vi "UHR-Fleezers Control (host) - 10.2.vi"() -> ()   [LabVIEW 2009] (continued)
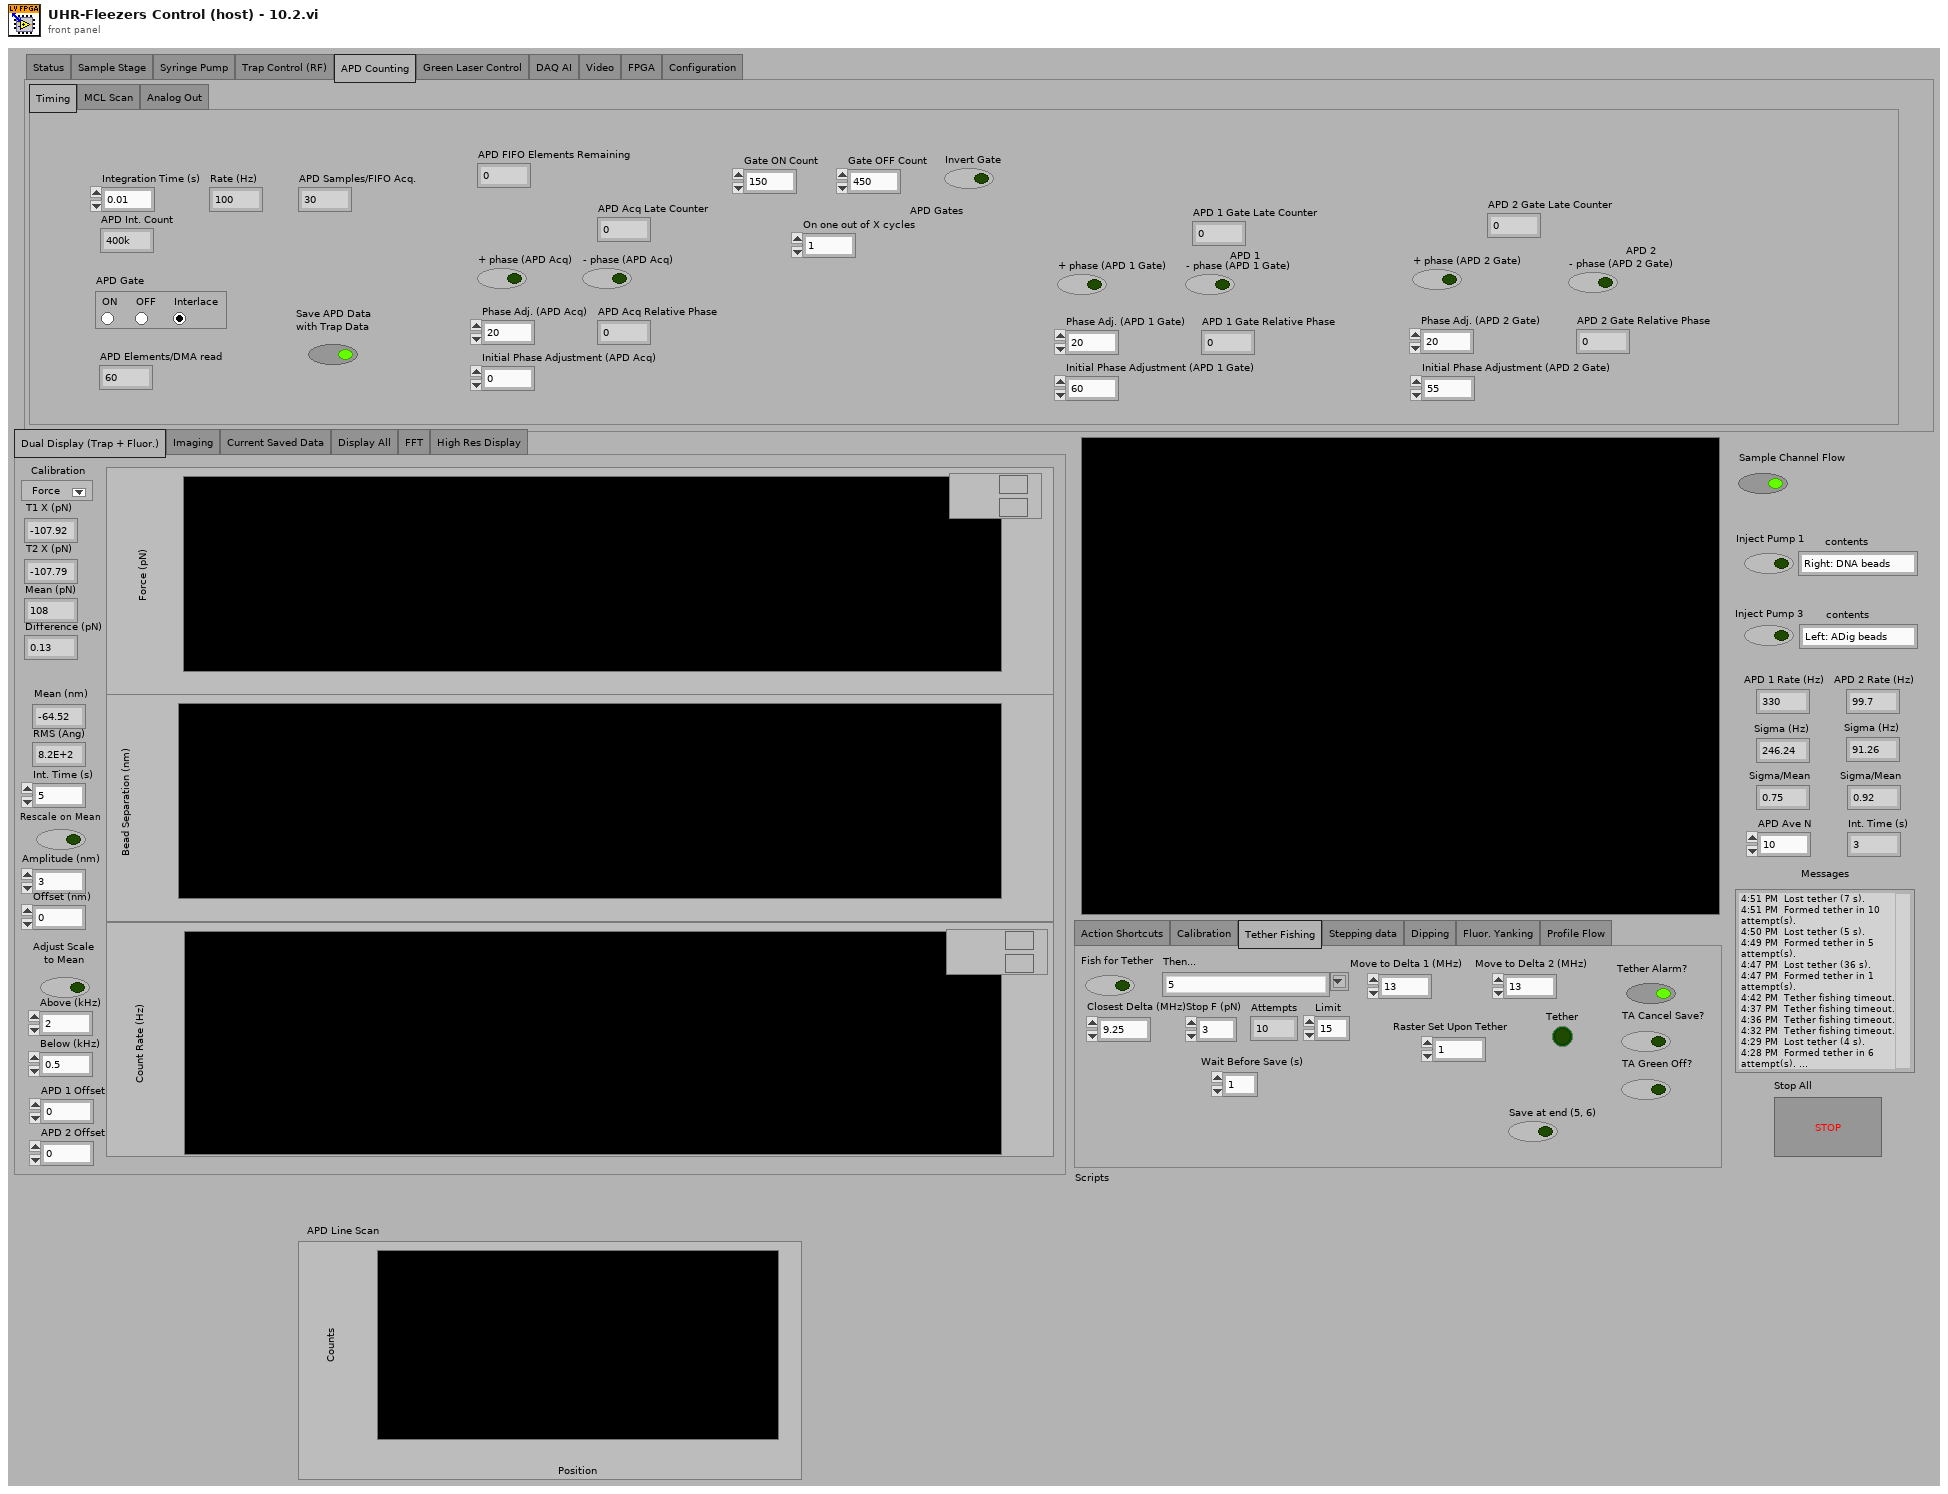
[diagram p1: front panel]
types:
  T1 = enum32{"Action Shortcuts", "Calibration", "Tether Fishing", "Stepping data", "Dipping", "Fluor. Yanking", "Profile Flow"}
  T2 = typedef "IMAQ Image.ctl" = refnum<image>
  T3 = enum32{"Dual Display (Trap + Fluor.)", "Imaging", "Current Saved Data", "Display All", "FFT", "High Res Display"}
  T4 = enum32{"Status", "Sample Stage", "Syringe Pump", "Trap Control (RF)", "APD Counting", "Green Laser Control", "DAQ AI", "Video", "FPGA", "Configuration"}
  T5 = cluster{"Pump 1":cluster{"Diameter (mm)":dbl, "Units":dbl, "Volume":dbl, "Rate":dbl}, "Pump 2":cluster{"Diameter (mm)":dbl, "Units":dbl, "Volume":dbl, "Rate":dbl}, "Pump 3":cluster{"Diameter (mm)":dbl, "Units":dbl, "Volume":dbl, "Rate":dbl}}
  T6 = enum32{"IR Laser Interlacing (Direct RF Board Control Method)", "AOD Raster Scan", "Feedback on Trap Intensity", "Feedback on Trap Position"}
  T7 = typedef "LVPoint32TypeDef.ctl" = cluster{"Horizontal":i32, "Vertical":i32}
  T8 = cluster{"Scan Range AOD (nm) 2":dbl, "Step Size AOD (nm) 2":dbl, "Scan Speed AOD (nm/s) 2":dbl, "Number of scans (AOD) 2":u16, "Label":string}[]
  T9 = cluster{"Set 1":cluster{"proportional gain (Kc)":i16, "integral gain (Kc*Ts/Ti)":i16, "derivative gain (Kc*Td/Ts)":i16}, "Set 2":cluster{"proportional gain (Kc)":i16, "integral gain (Kc*Ts/Ti)":i16, "derivative gain (Kc*Td/Ts)":i16}}
  T10 = cluster{"Trap 1":fxp<+/-,16,1>, "Trap 2":fxp<+/-,16,1>}
  T11 = cluster{"proportional gain (Kc)":fxp<+/-,16,8>, "integral gain (Kc*Ts/Ti)":fxp<+/-,16,8>, "derivative gain (Kc*Td/Ts)":fxp<+/-,16,8>}
  T12 = cluster{"output high":fxp<+/-,16,1>, "output low":fxp<+/-,16,1>}
  T13 = cluster{"Set 1":fxp<+/-,16,1>, "Set 2":fxp<+/-,16,1>}
  T14 = cluster{"proportional gain (Kc)":i16, "integral gain (Kc*Ts/Ti)":i16, "derivative gain (Kc*Td/Ts)":i16}
  T15 = cluster{"Set 1":bool, "Set 2":bool, "Set 3":bool}
  T16 = typedef "LVMinMaxIncTypeDef.ctl" = cluster{"Minimum":dbl, "Maximum":dbl, "Increment":dbl}
  T17 = typedef "Image Type" = u32
  T18 = typedef "nirio_resource_hc.ctl" = tag
  T19 = typedef "niFpgaNodeNameForErrorReporting.ctl" = enum16{"Open FPGA VI Reference", "Read/Write Control", "Invoke Method: Abort", "Invoke Method: Acknowledge IRQ", "Invoke Method: Download", "Invoke Method: FIFO.Configure", "Invoke Method: FIFO.Read", "Invoke Method: FIFO.Start", "Invoke Method: FIFO.Stop", "Invoke Method: FIFO.Write", "Invoke Method: Reset", "Invoke Method: Run", "Invoke Method: Wait on IRQ", "Close FPGA VI Reference"}
  T20 = typedef "niLvFpgaWhatHappensToTopLevelVI.ctl" = enum16{"top level VI scripted behind XNode", "top level VI inlined behind XNode"}
  T21 = typedef "openfpgaref.8.6.ctl" = refnum<k20>
  T22 = cluster{"New Image":T2, "New Image":T2, "New Image":T2, "New Image":T2}
  T23 = typedef "XDNodeRunTimeDep.lvlib/timing_clust.ctl" = cluster{"Expected End [f-1]":u64, "Actual End [f-1]":u64, "Finished Late? [f-1]":bool, "Expected End [i-1]":u64, "Actual End [i-1]":u64, "Finished Late? [i-1]":bool, "Expected Start [i]":u64, "Actual Start [i]":u64, "Expected Start [f]":u64, "Actual Start [f]":u64, "Source Name":string, "Structure Name":string, "Period":i64, "Deadline":i64, "Offset":i64, "Start":i64, "Priority":i32, "Timeout":i32, "Mode":T24, "Wakeup Reason":T25, "Error":errorcluster, "Source Type":string, "Secondary Source Type":string, "Global End Time":u64, "Global Start Time":u64, "Frame Duration":u64, "Iteration Duration":u64, "Assigned CPU":i32, "I/O Scan Engine Mode":u32}
  T24 = typedef "XDNodeRunTimeDep.lvlib/nitl_modes.ctl" = enum32{"No Change", "Process missed periods, maintain original phase", "Discard missed periods, maintain original phase", "Process missed periods, ignore original phase", "Discard missed periods, ignore original phase"}
  T25 = typedef "XDNodeRunTimeDep.lvlib/wakeup.ctl" = enum32{"Normal", "Aborted", "Asynchronous wakeup", "Timing source error", "Timed loop error", "Timeout"}
  T26 = enum32{"Normal Display", "Dual Display (APD)", "FFT", "High Res Display"}
  T27 = cluster{"Origin Pixel":cluster{"X":sgl, "Y":sgl}, "Angle Relative to Horizontal (deg)":sgl, "Axis Reference":u32}
  T28 = typedef "Simple Grid Descriptor" = cluster{"X Step":sgl, "Y Step":sgl, "Unit":T29}
  T29 = typedef "Image Unit" = enum32{"Undefined", "Angström", "Micrometer", "Millimeter", "Centimeter", "Meter", "Kilometer", "Microinch", "Inch", "Feet", "Nautical miles", "Standard miles", "Steps"}
  T30 = cluster{"averaging mode":u16, "weighting mode":u16, "number of averages":u32}
  T31 = cluster{"dB On (F)":bool, "unwrap phase (F)":bool, "convert to degree (F)":bool}
  T32 = cluster{"Green FB Ch 0":i16, "Green FB Ch 1":i16, "Green FB Ch 2":i16}
  T33 = enum16{"open", "replace", "create", "open or create", "replace or create", "replace or create with confirmation"}
  T34 = enum16{"big-endian, network order", "native, host order", "little-endian"}
  T35 = cluster{string, string, string, string, string, string, string, string}
  T36 = cluster{string, string, string, string, string, string, string, string, string, string, string, string}
  T37 = cluster{string, string, string, string, string, string, string, string, string, string, string, string, string}
  T38 = cluster{string, string, string, string, string, string, string, string, string, string, string, string, string, string}
  T39 = cluster{"BD 1 Frequency 1 (MHz)":dbl, "BD 1 Frequency 2 (MHz)":dbl}
  T40 = cluster{"f0":dbl, "df":dbl, "magnitude":dbl[]}[][]
  T41 = cluster{"Green FB Ch 0":dbl, "Green FB Ch 1":dbl, "Green FB Ch 2":dbl}
  T42 = cluster{"Scan Range AOD (nm) 2":dbl, "Step Size AOD (nm) 2":dbl, "Scan Speed AOD (nm/s) 2":dbl, "Number of scans (AOD) 2":u16, "Label":string}
  T43 = cluster{"[0]":dbl, "[1]":dbl, "[2]":dbl, "[3]":dbl, "[4]":dbl, "[5]":dbl}
  T44 = cluster{"Diameter (mm)":dbl, "Units":dbl, "Volume":dbl, "Rate":dbl}
  T45 = cluster{"Left":i32, "Top":i32, "Width":u32, "Height":u32}
  T46 = cluster{cluster{"Left":i32, "Top":i32, "Width":u32, "Height":u32}}[]
  T47 = enum32{"setting", "request", "request control", "info", "statistics", "system settings", "I/O sub system", "HRT control", "camera descriptions", "device specific data", "event sub system settings", "event sub system results", "image memory manager"}
  T48 = typedef "AviRefnum.ctl" = refnum<k1>
  T49 = typedef "imagedata.ctl" = cluster{"image type":i32, "image depth":i32, "image":u8[], "mask":u8[], "colors":u32[], "Rectangle":cluster{"left":i16, "top":i16, "right":i16, "bottom":i16}}
diagram:
  w25 = u16 20 items=["1.0"=10, "1.5"=15, "2.0"=20] ("stop bits (10: 1 bit)")
  w32 = T17 2 items=["Grayscale (U8)", "Grayscale (I16)", "Grayscale (SGL)", "Complex (CSG)", "RGB (U32)", "HSL (U32)", "RGB (U64)", "Grayscale (U16)"] ("Image Type")
  w100 = cluster{"output high":i16, "output low":i16} {"output high"=3000, "output low"=0} ("FB output range 1")
  w182 = 10.0 ("y")
  w181 = 32767.0 ("y")
  w197 = 6.0  # clock mult.
  w198 = 49152000.0  # TCXO frequ.
  n1 = Build Array("DIO count 1 (ticks)", "DIO count 2 (ticks)", "DIO count 3 (ticks)") -> (w87:u32[])
  n2 = Multiply(x="APD Integration Time (s)", y=40000000.0) -> (x*y=w107:dbl)
  n3 = Reciprocal(x="APD Integration Time (s)") -> (1/x=w104:dbl)
  n4 = local write "APD Acq Rate (Hz)"(w104) -> ()
  n5 = local read "AO1"() -> (w176:dbl)
  n6 = local read "AO2"() -> (w175:dbl)
  n7 = To Unsigned Long Integer(number=w107) -> (unsigned 32bit integer=w106:u32)
  "APD Int. Count" <- w106
  n8 = local read "Scan Increment (MHz)"() -> (w193:dbl)
  n9 = local read "Continuous MCL Scanning"() -> (w163:bool)
  n10 = local read "Fast Scan Dir"() -> (w162:bool)
  n11 = Multiply(x=w176, y=w181) -> (x*y=w178:dbl)
  n12 = local read "Number of scans (MCL)"() -> (w164:u64)
  n13 = Multiply(x=w175, y=w181) -> (x*y=w180:dbl)
  n14 = Divide(x=w178, y=w182) -> (x/y=w177:dbl)
  n15 = Divide(x=w180, y=w182) -> (x/y=w179:dbl)
  n16 = To Word Integer(number=w177) -> (16bit integer=w174:i16)
  n17 = To Word Integer(number=w179) -> (16bit integer=w173:i16)
  n18 = Not(x=w162) -> (.not. x?=w157:bool)
  n19 = local read "Cycles/step (MCL)"() -> (w165:u64)
  n20 = Multiply(x=w193, y=1000.0) -> (x*y=w200:dbl)
  n21 = local read "Scan steps (MCL)"() -> (w166:u64)
  n22 = local write "Trap Pos FIFO Timeout"(u16 0 ("Trap Pos FIFO Timeout")) -> ()
  n23 = local read "Desired Scan Incr (V)"() -> (w168:dbl)
  n24 = Scale By Power Of 2(n=48, x=w200) -> (x*2^n=w201:dbl)
  n25 = Multiply(x=w198, y=w197) -> (x*y=w196:dbl)
  n26 = Divide(x=w201, y=w196) -> (x/y=w195:dbl)
  n27 = local read "Setpoints (V)"() -> (w215:cluster{"Set 1":dbl, "Set 2":dbl})
  n28 = property on="AI Count (ticks)" class="DigNum (strict)"("Val(Sgnl)"="AI Count (ticks)") -> ()  [unwired: 2 in, 2 out]
  n29 = local read "Number Interlace Sets"() -> (w80:u8)
  n30 = Split 1D Array(array=w87, index=w80) -> (first subarray=w89:u32[])  [unwired: 1 out]
  n31 = Add Array Elements(numeric array=w89) -> (sum=w88:u32)
  n32 = local read "# Samples/channel"() -> (w185:u32)
  n33 = To Quad Integer(1:w195) -> (0:w192:i64)
  n34 = local read "Number of F/B Scans (AOD)"() -> (w186:u16)
  n35 = local read "Not-Interlacing Set"() -> (w79:enum32{"Set 1", "Set 2", "Set 3"})
  n36 = To Unsigned Byte Integer(number=w79) -> (unsigned 8bit integer=w85:u8)
  n37 = Index Array(array=w87, index=w85) -> (element=w86:u32)
  n38 = Divide(x=40000000.0, y="AI Count (ticks)") -> (x/y=w153:dbl)
  n39 = Multiply(x=w168, y=32767.0) -> (x*y=w170:dbl)
  n40 = local read "Feedback On/Off"() -> (w218:cluster{"Set 1":bool, "Set 2":bool})
  n41 = local read "PID Gains"() -> (w210:T9)
  n42 = local read "Scan steps (AOD)"() -> (w191:u64)
  n43 = local read "All FB On/Off"() -> (w219:bool)
  n44 = local read "Cycles/step (AOD)"() -> (w190:u64)
  n45 = local write "AI rate (Hz)"(w153) -> ()
  n46 = Divide(x=w170, y=10.0) -> (x/y=w169:dbl)
  n47 = Multiply(x=w191, y=w190) -> (x*y=w189:u64)
  n48 = Multiply(x=3276.7, y=w215) -> (x*y=w214:cluster{"Set 1":dbl, "Set 2":dbl})
  n49 = To Word Integer(number=w169) -> (16bit integer=w167:i16)
  n50 = Multiply(x=w189, y=u64 2) -> (x*y=w187:u64)
  n51 = Divide(x=w153, y="FPGA Ave.") -> (x/y=w154:dbl)
  n52 = To Word Integer(number=w214) -> (16bit integer=w213:cluster{"Set 1":i16, "Set 2":i16})
  n53 = xnode "Open FPGA VI Reference"("resource name"=T18 "750kHzDAQ") -> ("FPGA VI Reference Out"=w207:refnum<k20>, "error out"=w206:errorcluster)  [unwired: 1 in]
  n54 = local read "Sets to FIFO (Traps)"() -> (w222:T15)
  n55 = Unbundle By Name(w210) -> ("Set 1"=w209:T14, "Set 2"=w208:T14)
  n56 = Multiply(x=w187, y=w186) -> (x*y=w184:u64)
  n57 = Divide(x=w184, y=w185) -> (x/y=w183:dbl)
  n58 = local write "Ave. Rate (Hz)"(w154) -> ()
  n59 = Unbundle By Name(w213) -> ("Set 1"=w212:i16, "Set 2"=w211:i16)
  n60 = local read "2D or 1D Scan"() -> (w101:bool)
  n61 = local write "Data points/scans"(w184) -> ()
  n62 = And(x=w218, y=w219) -> (x .and. y?=w217:cluster{"Set 1":bool, "Set 2":bool})
  n63 = local read "Scan BD"() -> (w202:bool)
  n64 = Reciprocal(x=w154) -> (1/x=w155:dbl)
  n65 = local write "Data points/scan (f/b)"(w187) -> ()
  n66 = local read "N Acq Sets (Traps + Fl.)"() -> (w146:i16)
  n67 = local write "N sets should be saved"(w183) -> ()
  n68 = Unbundle By Name(w217) -> ("Set 1"=w221:bool, "Set 2"=w220:bool)
  n69 = xnode "Invoke Method"("FPGA VI Reference In"=w207, "error in"=w206) -> ("FPGA VI Reference Out"=w99:refnum<k20>, "error out"=w120:errorcluster)
  n70 = local read "Interlace"() -> (w81:bool)
  n71 = Select(t=w88, s=w81, f=w86) -> (s? t:f=w78:u32)
  n72 = local write "Update Count (MCL)"(w78) -> ()
  n73 = local write "Total Counts (ticks)"(w78) -> ()
  n74 = local write "Ave. Period (s)"(w155) -> ()
  n75 = property on="2D or 1D Scan" class="Bool (strict)"("Val(Sgnl)"=w101) -> ()  [unwired: 2 in, 2 out]
  n76 = xnode "Read/Write Control"("FPGA VI Reference In"=w98, "error in"=w120, "ai count"="AI Count (ticks)", "Interlace ON/OFF"=w81, "Number Interlace Cycles"=w80, "AI1 Sets to FIFO"=w222, "FB On/Off Set 1"=w221, "FB On/Off Set 2"=w220, "Interlace Off Parameters"=w79, "FB Setpoint Set 1"=w212, "FB Setpoint Set 2"=w211, "FB Gains Set 1"=w209, "FB Gains Set 2"=w208, "FB output range 1"=w100, "FB output range 2"=w100, "Cycles per step"=w190, "Scan BD"=w202, "Number of scans"=w186, "Scan steps"=w191, "Scan freq.  increment"=w192, "AO1"=w174, "AO2"=w173, "Scan freq.  increment (MCL)"=w167, "Scan steps (MCL)"=w166, "Cycles per step (MCL)"=w165, "Number of scans (MCL)"=w164, "MCL count"=w78, "Cont. Scan (MCL)"=w163, "MCL Scan Axis"=w157, "1D or 2D Scan?"=w101, "N of AI1 Int Acq Sets"=w146, "Freq or Amp switch first"="Freq or Amp switch first", "Freq switch delay"="Freq switch delay", "Amp switch delay"="Amp switch delay", "Swap F1 and F2"="Swap F1 and F2", "APD Acq Rate Count"=w106, "APD to FIFO"=FALSE, "APD Gate Operating Mode"="APD Gate", "APD Gate ON Count"="APD Gate ON Count", "APD Gate OFF Count"="APD Gate OFF Count", "Invert APD Gate"="Invert APD Gate", "DIO count 1 (ticks)"="DIO count 1 (ticks)", "DIO count 2 (ticks)"="DIO count 2 (ticks)", "DIO count 3 (ticks)"="DIO count 3 (ticks)", "APD 1 AO scale factor"="APD 1 AO Mult.", "APD 2 AO scale factor"="APD 2 AO Mult.") -> ("FPGA VI Reference Out"=w73:refnum<k20>, "error out"=w75:errorcluster)  [unwired: 1 in]
  n77 = local read "Green Laser ON/Interlacing"() -> (w76:bool)
  n78 = local read "Green laser mode"() -> (w77:enum32{"Laser ON", "Laser OFF", "Interlace"})
  n79 = local read "GI Frequency, OFF count"() -> (w69:u32)
  n80 = local read "GI Frequency, ON count"() -> (w68:u32)
  n81 = Multiply(x="Current When FB OFF (%)", y=655.35) -> (x*y=w59:dbl)
  n82 = local read "Green FB Count"() -> (w67:u32)
  n83 = Multiply(x="Green FB Setpoint (mV)", y=3.2767) -> (x*y=w56:dbl)
  n84 = To Unsigned Word Integer(number=w59) -> (unsigned 16bit integer=w57:u16)
  n85 = local read "Invert GI"() -> (w71:bool)
  n86 = To Word Integer(number=w56) -> (16bit integer=w54:i16)
  n87 = case shown="False" w76 {
    tunnel: w77 -> [_ w248]
    tunnel: [enum32{"Laser ON", "Laser OFF", "Interlace"}."Laser OFF" ("Green laser mode") w248] -> w70
    frame #0 {
    }
    frame #1 {
    }
  }
  n88 = local read "Trap Pos. AI1 X Pre-scale"() -> (w11:u16)
  n89 = local read "Trap Pos FB Monitor\nT1 or T2"() -> (w18:bool)
  n90 = local read "Trap Pos FB Int Count"() -> (w4:u16)
  n91 = local read "Trap Pos FB Negate Action"() -> (w17:bool)
  n92 = local read "Trap Pos. FB Offset Factor"() -> (w16:i64)
  n93 = local read "Trap Pos. FB Mult Factor"() -> (w15:i64)
  n94 = local read "Trap Pos. FB Gains"() -> (w13:T11)
  n95 = local read "Trap Pos. FB Range"() -> (w14:T12)
  n96 = xnode "Read/Write Control"("FPGA VI Reference In"=w73, "error in"=w75, "Green interlace ON count 2"=w68, "Green interlace OFF count 2"=w69, "Invert GI 2"=w71, "Operating Mode 2"=w70, "Green FB Gains"="Green FB Gains", "Green FB Setpoint"=w54, "Green FB On/Off"="Green FB On/Off", "Current Out"=w57, "Green int current ON count adj"="Green int current ON count adj", "Green FB Count"=w67, "Operating Mode"=w70, "Green interlace OFF count"=w69, "Green interlace ON count"=w68, "Invert GI"=w71, "Trap Pos FB Monitor T1 or T2"=w18, "Trap Pos FB Negate Action"=w17, "Trap Pos. FB Offset Factor"=w16, "Trap Pos. FB Mult Factor"=w15, "Trap Pos. FB Range"=w14, "Trap Pos. FB Gains"=w13, "Force feedback"=FALSE, "AI1 X Scale"=w11, "Trap Pos to FIFO"=TRUE, "Trap Pos FB Int Count"=w4) -> ("FPGA VI Reference Out"=w72:refnum<k20>, "error out"=w74:errorcluster)
  n97 = xnode "Invoke Method"("FPGA VI Reference In"=w72, "error in"=w74, "Depth"="Trap AI FIFO Depth") -> ("FPGA VI Reference Out"=w21:refnum<k20>, "error out"=w20:errorcluster)
  n98 = xnode "Invoke Method"("FPGA VI Reference In"=w21, "error in"=w20, "Depth"="Trap Position FIFO Depth") -> ("FPGA VI Reference Out"=w6:refnum<k20>, "error out"=w5:errorcluster)
  n99 = flat-sequence {
    tunnel: w99 -> [w253]
    tunnel: [w253] -> w98
    tunnel: [w252] -> w97
    tunnel: [w251] -> w96
    tunnel: [w249] -> w94
    tunnel: [w250] -> w95
    frame #0 {
      w250 = T16 {"Minimum"=0.0, "Maximum"=40.0, "Increment"=1.0} ("Min Max Inc")
      w249 = T16 {"Minimum"=0.0, "Maximum"=50.0, "Increment"=1.0} ("Data Entry Limits")
      w252 = T16 {"Minimum"=60.0, "Maximum"=90.0, "Increment"=1.0} ("Min Max Inc")
      w251 = T16 {"Minimum"=0.0, "Maximum"=50.0, "Increment"=1.0} ("Data Entry Limits")
      n100 = property on="BD 2 Frequency 1 (MHz)" class="DigNum (strict)"("Data Range"=w250) -> ()  [unwired: 2 in, 2 out]
      n101 = property on="BD 2 Frequency 3 (MHz)" class="DigNum (strict)"("Data Range"=w250) -> ()  [unwired: 2 in, 2 out]
      n102 = property on="BD 2 Frequency 2 (MHz)" class="DigNum (strict)"("Data Range"=w250) -> ()  [unwired: 2 in, 2 out]
      n103 = property on="BD 1 Frequency 1 (MHz)" class="DigNum (strict)"("Data Range"=w252) -> ()  [unwired: 2 in, 2 out]
      n104 = property on="BD 1 Frequency 2 (MHz)" class="DigNum (strict)"("Data Range"=w252) -> ()  [unwired: 2 in, 2 out]
      n105 = property on="BD 1 Frequency 3 (MHz)" class="DigNum (strict)"("Data Range"=w252) -> ()  [unwired: 2 in, 2 out]
      n106 = property on="BD 2 Amplitude 1 (%)" class="DigNum (strict)"("Data Range"=w249) -> ()  [unwired: 2 in, 2 out]
      n107 = property on="BD 2 Amplitude 2 (%)" class="DigNum (strict)"("Data Range"=w249) -> ()  [unwired: 2 in, 2 out]
      n108 = property on="BD 2 Amplitude 3 (%)" class="DigNum (strict)"("Data Range"=w249) -> ()  [unwired: 2 in, 2 out]
      n109 = property on="BD 1 Amplitude 3 (%)" class="DigNum (strict)"("Data Range"=w251) -> ()  [unwired: 2 in, 2 out]
      n110 = property on="BD 1 Amplitude 2 (%)" class="DigNum (strict)"("Data Range"=w251) -> ()  [unwired: 2 in, 2 out]
      n111 = property on="BD 1 Amplitude 1 (%)" class="DigNum (strict)"("Data Range"=w251) -> ()  [unwired: 2 in, 2 out]
      "X RF Frequency Limits (MHz)" <- w252
      "X RF Amplitude Limits (%)" <- w251
      "Y RF Amplitude Limits (%)" <- w249
      "Y RF Frequency Limits (MHz)" <- w250
    }
  }
  n112 = xnode "Invoke Method"("FPGA VI Reference In"=w6, "error in"=w5) -> ("FPGA VI Reference Out"=w119:refnum<k20>, "error out"=w118:errorcluster)  [unwired: 1 out]
  n113 = flat-sequence "Initial FPGA Loop Relative Phase Adjustment" {
    tunnel: "Initial Phase Adjustment (AI1)" -> [w264]
    tunnel: "Initial Phase Adjustment (GI)" -> [w263]
    tunnel: w119 -> [w262]
    tunnel: w118 -> [w261]
    tunnel: "Initial Phase Adj. (MCL)" -> [w260]
    tunnel: [w265] -> w128
    tunnel: [w259] -> w124
    tunnel: "Initial Phase Adjustment (APD Acq)" -> [w258]
    tunnel: "Initial Phase Adjustment (APD 1 Gate)" -> [w257]
    tunnel: "Initial Phase Adjustment (Green FB)" -> [w256]
    tunnel: "Initial Phase Adjustment (GI) 2" -> [w255]
    tunnel: "Initial Phase Adjustment (APD 2 Gate)" -> [w254]
    tunnel: w128 -> [w436]
    tunnel: [w437] -> w125
    tunnel: w124 -> [w437]
    tunnel: [w436] -> w123
    tunnel: w125 -> [w440]
    tunnel: w123 -> [w439]
    tunnel: [w442] -> w122
    tunnel: [w441] -> w121
    tunnel: [w621] -> w126
    tunnel: [w622] -> w127
    tunnel: w122 -> [w622]
    tunnel: w121 -> [w621]
    frame #0 {
      n114 = xnode "Read/Write Control"("FPGA VI Reference In"=w262, "error in"=w261, "Phase count adjustment"=w264, "Phase count adjustment (GI)"=w263, "Phase count adjustment (MCL)"=w260, "Phase Count Adjustment (APD Acq)"=w258, "Phase count adjustment (APD 1 Gate)"=w257, "Phase count adjustment (APD 2 Gate)"=w254, "Phase count adjustment (Green FB)"=w256, "Phase count adjustment (GI) 2"=w255) -> ("FPGA VI Reference Out"=w259:refnum<k20>, "error out"=w265:errorcluster)
    }
    frame #1 {
      n115 = Wait (ms)(milliseconds to wait=u32 100) -> ()  [unwired: 1 out]
    }
    frame #2 {
      w438 = TRUE
      n116 = xnode "Read/Write Control"("FPGA VI Reference In"=w440, "error in"=w439, "+ phase"=w438, "+ phase (GI)"=w438, "+ phase (MCL)"=w438, "+ phase (APD Acq)"=w438, "+ phase (APD 1 Gate)"=w438, "+ phase (APD 2 Gate)"=w438, "+ phase (Green FB)"=w438, "+ phase (GI) 2"=w438) -> ("FPGA VI Reference Out"=w441:refnum<k20>, "error out"=w442:errorcluster)
    }
    frame #3 {
      n117 = Wait (ms)(milliseconds to wait=u32 100) -> ()  [unwired: 1 out]
    }
  }
  n118 = local read "Phase adj. (Green FB)"() -> (w90:i16)
  n119 = local read "Phase adj. (GI) 2"() -> (w60:i16)
  n120 = local read "Phase adjust (MCL)"() -> (w158:i16)
  n121 = local read "Phase adj. (AI1)"() -> (w160:i16)
  n122 = local read "Phase adj. (GI)"() -> (w159:i16)
  n123 = xnode "Read/Write Control"("FPGA VI Reference In"=w126, "error in"=w127, "Phase count adjustment"=w160, "Phase count adjustment (GI)"=w159, "Phase count adjustment (MCL)"=w158, "Phase Count Adjustment (APD Acq)"="Phase Adj. (APD Acq)", "Phase count adjustment (APD 1 Gate)"="Phase Adj. (APD 1 Gate)", "Phase count adjustment (APD 2 Gate)"="Phase Adj. (APD 2 Gate)", "Phase count adjustment (Green FB)"=w90, "Phase count adjustment (GI) 2"=w60) -> ("FPGA VI Reference Out"=w46:refnum<k20>, "error out"=w135:errorcluster)
  n124 = call "Initialize RF boards - interlace 3.vi"("error in"=w135, "FPGA VI Reference In"=w46) -> ("error out"=w133:errorcluster, "FPGA VI Reference Out"=w134:T21)
  n125 = call "set RF board frequency - interlace.vi"("Board 2 Frequency Limits"=w95, "Board 1 Frequency Limits"=w97, "error in"=w133, "FPGA VI Reference In"=w134, "Board 2 Frequency 3 (MHz)"="BD 2 Frequency 3 (MHz)", "Board 1 Frequency 3 (MHz)"="BD 1 Frequency 3 (MHz)", "Board 2 Frequency 2 (MHz)"="BD 2 Frequency 2 (MHz)", "Board 2 Frequency 1 (MHz)"="BD 2 Frequency 1 (MHz)", "Board 1 Frequency 2 (MHz)"="BD 1 Frequency 2 (MHz)", "Board 1 Frequency 1  (MHz)"="BD 1 Frequency 1 (MHz)") -> ("error out"=w237:errorcluster, "FPGA VI Reference Out"=w238:T21)
  n126 = call "set RF board amplitude - interlace.vi"("Board 2 Amplitude Limits"=w94, "Board 1 Amplitude Limits"=w96, "error in"=w237, "FPGA VI Reference In"=w238, "Board 2 Amplitude 3 (%)"="BD 2 Amplitude 3 (%)", "Board 1 Amplitude 3 (%)"="BD 1 Amplitude 3 (%)", "Board 2 Amplitude 2 (%)"="BD 2 Amplitude 2 (%)", "Board 2 Amplitude 1 (%)"="BD 2 Amplitude 1 (%)", "Board 1 Amplitude 2 (%)"="BD 1 Amplitude 2 (%)", "Board 1 Amplitude 1 (%)"="BD 1 Amplitude 1 (%)") -> ("error out"=w225:errorcluster, "FPGA VI Reference Out"=w226:T21)
  n127 = flat-sequence {
    tunnel: w226 -> [w631]
    tunnel: w225 -> [w630]
    tunnel: [w629] -> w230
    tunnel: [w628] -> w229
    tunnel: [w672] -> w228
    tunnel: w230 -> [w672]
    tunnel: [w671] -> w227
    tunnel: w229 -> [w671]
    tunnel: w228 -> [w681]
    tunnel: w227 -> [w680]
    tunnel: [w679] -> w8
    tunnel: [w678] -> w7
    frame #0 {
      n128 = local read "Trap 1 (ON/OFF)"() -> (w623:bool)
      n129 = xnode "Read/Write Control"("FPGA VI Reference In"=w631, "error in"=w630, "Direct RF Box  Communication"=FALSE) -> ("FPGA VI Reference Out"=w629:T21, "error out"=w628:errorcluster)
      n130 = local write "Saving..."(FALSE ("Saving Data")) -> ()
      n131 = local write "Stop All"(FALSE ("Stop All")) -> ()
      n132 = local write "Index"(1.0 ("Index")) -> ()
      n133 = property on="Trap 1 ON" class="Bool (strict)"("Value"=w623) -> ()  [unwired: 2 in, 2 out]
      "Manipulating Trap" <- FALSE ("Manipulating Trap")
    }
    frame #1 {
      n134 = local read "Trap 2 (ON/OFF)"() -> (w670:bool)
      n135 = Wait (ms)(milliseconds to wait=u32 10) -> ()  [unwired: 1 out]
      n136 = property on="Trap 2 ON" class="Bool (strict)"("Val(Sgnl)"=w670) -> ()  [unwired: 2 in, 2 out]
    }
    frame #2 {
      n137 = local read "Scan Range (nm)"() -> (w674:dbl)
      n138 = xnode "Read/Write Control"("FPGA VI Reference In"=w681, "error in"=w680, "FPGA Controls  RF Box"=TRUE ("Direct RF Box  Communication")) -> ("FPGA VI Reference Out"=w679:T21, "error out"=w678:errorcluster)
      n139 = call "Update messages.vi"("Message to add"="UHR-Fleezers ready.", "Old message string"="") -> ("New message string"=w677:string)
      n140 = property on="Scan Range (nm)" class="DigNum (strict)"("Val(Sgnl)"=w674) -> ()  [unwired: 2 in, 2 out]
      n141 = local write "Messages"(w677) -> ()
    }
  }
  n142 = Subtract(x="BD 1 Frequency 1 (MHz)", y="BD 1 Frequency 2 (MHz)") -> (x-y=w145:dbl)
  n143 = Subtract(x="BD 2 Frequency 1 (MHz)", y="BD 2 Frequency 2 (MHz)") -> (x-y=w144:dbl)
  n144 = Square(x=w144) -> (x^2=w142:dbl)
  n145 = Square(x=w145) -> (x^2=w143:dbl)
  n146 = Add(x=w143, y=w142) -> (x+y=w141:dbl)
  n147 = Square Root(x=w141) -> (sqrt(x)=w140:dbl)
  n148 = local write "Trap Delta (MHz)"(w140) -> ()
  n149 = call-poly "VISA Configure Serial Port"("VISA resource name"="Sample Chamber Stage Serial Port") -> ("VISA resource name out"=w41:refnum<visa-resource-name>, "error out"=w42:errorcluster)  [unwired: 5 in, 8 out]
  "Stage Control Serial Error" <- w42
  n150 = call "IMAQ Create"("Image Name"="APD 1 Image", "Image Type"=w32) -> ("New Image"=w31:T2)  [unwired: 3 in, 1 out]
  n151 = call "IMAQ Create"("Image Name"="APD 2 Image", "Image Type"=w32) -> ("New Image"=w30:T2)  [unwired: 3 in, 1 out]
  n152 = call "IMAQ Create"("Image Name"="Det. X Image", "Image Type"=w32) -> ("New Image"=w29:T2)  [unwired: 3 in, 1 out]
  n153 = call "IMAQ Create"("Image Name"="Det. Y Image", "Image Type"=w32) -> ("New Image"=w28:T2)  [unwired: 3 in, 1 out]
  n154 = call-poly "VISA Configure Serial Port"("VISA resource name"="Harvard Syringe Pump Serial Port", "baud rate (9600)"=u32 115200, "stop bits (10: 1 bit)"=w25) -> ("VISA resource name out"=w22:refnum<visa-resource-name>, "error out"=w23:errorcluster)  [unwired: 4 in, 7 out]
  n155 = Bundle("New Image"=w31, "New Image"=w30, "New Image"=w29, "New Image"=w28) -> (w27:T22)  [unwired: 1 in]
  n156 = node-c288(i64 1 ("Period"), 1 ("Processor")) -> (w149:T23)  [unwired: 2 out]
  n157 = node-c288(2 ("Processor")) -> (w50:T23)  [unwired: 3 out]
  n158 = node-c288() -> (w52:T23)  [unwired: 4 out]
  n159 = node-c288() -> (w37:T23)  [unwired: 4 in]
  n160 = node-c288(3 ("Processor")) -> (w48:T23)  [unwired: 3 out]
  n161 = timed-loop "Acquire Data" {
    tunnel: w8 -> [w971]
    tunnel: w7 -> [w970]
    tunnel: [w1001] -> w245
    tunnel: [w995] -> w243
    timing: w149 -> [_]
    timing-out: [_] -> w148
    tunnel: w27 -> [w796]
    stop <- "Stop All" stop-if-true
    w781 = "NI_ChannelName" ("name")
    n162 = node-c288() -> ()  [unwired: 2 out]
    n163 = First Call?() -> (First Call?: T/F=w746:bool)
    n164 = Or(x="Reset", y=w746) -> (x .or. y?=w747:bool)
    n165 = case "Reset data stream" shown="True" w747 {
      tunnel: w971 -> [w3250 w3258]
      tunnel: w970 -> [w3249 w3257]
      tunnel: [w3250 w3252] -> w966
      tunnel: [w3249 w3251] -> w965
      frame #0 {
      }
      frame #1 {
        w3255 = TRUE ("AI to FIFO")
        n166 = local write "Overflow (data lost)"(FALSE ("Overflow (data lost)")) -> ()
        n167 = call "reset FPGA DMA.vi"("error in"=w3257, "FPGA VI Reference In"=w3258) -> ("error out"=w3253:errorcluster, "FPGA VI Reference Out"=w3254:T21)
        n168 = xnode "Read/Write Control"("FPGA VI Reference In"=w3254, "error in"=w3253, "AI to FIFO"=w3255, "APD to FIFO"=w3255) -> ("FPGA VI Reference Out"=w3252:T21, "error out"=w3251:errorcluster)
      }
    }
    n169 = Or(x="Start AOD Scan", y="Trap Raster Scan") -> (x .or. y?=w916:bool)
    n170 = case "Start AOM raster scan" shown="True" w916 {
      tunnel: w966 -> [w2464 w2474]
      tunnel: w965 -> [w2463 w2473]
      tunnel: [w2464 w2467] -> w964
      tunnel: [w2463 w2466] -> w963
      frame #0 {
      }
      frame #1 {
        n171 = case shown="True" "Restart DMA? (AOD)" {
          tunnel: [w2840 w2842] -> w2468
          tunnel: [w2839 w2841] -> w2469
          tunnel: w2474 -> [w2840 w2844]
          tunnel: w2473 -> [w2839 w2843]
          frame #0 {
          }
          frame #1 {
            n172 = local write "Overflow (data lost)"(FALSE ("Overflow (data lost)")) -> ()
            n173 = call "reset FPGA DMA.vi"("error in"=w2843, "FPGA VI Reference In"=w2844) -> ("error out"=w2841:errorcluster, "FPGA VI Reference Out"=w2842:T21)
          }
        }
        n174 = local write "Trap Raster Scan"(FALSE ("Trap Raster Scan")) -> ()
        n175 = case shown="True" "Move MCL Also?" {
          tunnel: w2469 -> [w2477 w2583]
          tunnel: w2468 -> [w2478 w2584]
          tunnel: [w2476 w2587] -> w2467
          tunnel: [w2475 w2586] -> w2466
          frame #0 {
            w2479 = TRUE ("AI to FIFO")
            n176 = xnode "Read/Write Control"("FPGA VI Reference In"=w2478, "error in"=w2477, "AI to FIFO"=w2479, "APD to FIFO"=w2479, "Start scan"=w2479) -> ("FPGA VI Reference Out"=w2476:T21, "error out"=w2475:errorcluster)
          }
          frame #1 {
            w2580 = FALSE ("1D or 2D Scan?")
            w2585 = TRUE ("AI to FIFO")
            # "Count for MCL loop"
            # "N total cycles"
            # "N steps"
            # "V_int"
            n177 = local read "Scan Range (nm)"() -> (w2562:dbl)
            n178 = local read "Number of F/B Scans (AOD)"() -> (w2579:u16)
            n179 = Sign(1:w2562) -> (0:w2561:dbl)
            n180 = Compound Arithmetic op=MULTIPLY(w2562, "MCL Step Position Ratio", "MCL/AOM Scale Tweak") -> (w2566:dbl)
            n181 = Negate(x=w2561) -> (-x=w2558:dbl)
            n182 = Multiply(x=w2558, y="MCL Step Increment (V_int)") -> (x*y=w2560:dbl)
            n183 = Divide(x=w2566, y="MCL X Cal (nm/V)") -> (x/y=w2572:dbl)
            n184 = Multiply(x=32767.0 ("y"), y=w2572) -> (x*y=w2578:dbl)
            n185 = local read "Total Counts (ticks)"() -> (w2563:u32)
            n186 = local read "Cycles/step (AOD)"() -> (w2574:u64)
            n187 = local read "Scan steps (AOD)"() -> (w2575:u64)
            n188 = Divide(x=w2578, y=10.0) -> (x/y=w2571:dbl)
            n189 = Divide(x=w2571, y="MCL Step Increment (V_int)") -> (x/y=w2569:dbl)
            n190 = Absolute Value(x=w2569) -> (abs(x)=w2557:dbl)
            n191 = Compound Arithmetic op=MULTIPLY(w2575, w2574, w2563) -> (w2570:u64)
            n192 = local write "wait to reset values"(w2585) -> ()
            n193 = local write "MCL Scanning"(w2585) -> ()
            n194 = Divide(x=w2570, y=w2557) -> (x/y=w2567:dbl)
            "MCL Count" <- w2567
            n195 = xnode "Read/Write Control"("FPGA VI Reference In"=w2584, "error in"=w2583, "Scan steps (MCL)"=w2557, "Number of scans (MCL)"=w2579, "Cycles per step (MCL)"=u64 1, "Scan freq.  increment (MCL)"=w2560, "1D or 2D Scan?"=w2580, "MCL Scan Axis"=w2580, "Cont. Scan (MCL)"=w2580, "MCL count"=w2567) -> ("FPGA VI Reference Out"=w2582:T21, "error out"=w2581:errorcluster)
            n196 = xnode "Read/Write Control"("FPGA VI Reference In"=w2582, "error in"=w2581, "AI to FIFO"=w2585, "APD to FIFO"=w2585, "Start scan"=w2585, "Start scan (MCL)"=w2585) -> ("FPGA VI Reference Out"=w2587:T21, "error out"=w2586:errorcluster)
          }
        }
        "Raster Scanning..." <- TRUE ("Scanning...")
      }
    }
    n197 = And(x="Save scans", y=w916) -> (x .and. y?=w962:bool)
    n198 = Compound Arithmetic op=OR("Start MCL Scan", "Confocal Image", "Confocal Linescan") -> (w914:bool)
    n199 = And(x="Save Data (MCL)", y=w914) -> (x .and. y?=w961:bool)
    n200 = case "Start MCL raster scan" shown="True" w914 {
      tunnel: w964 -> [w1816 w1831]
      tunnel: w963 -> [w1815 w1830]
      tunnel: [w1816 w1826] -> w794
      tunnel: [w1815 w1825] -> w793
      tunnel: [FALSE w1824] -> w947
      tunnel: "Start MCL Scan" -> [_ w1819]
      tunnel: "Confocal Image" -> [_ w1818]
      tunnel: "Confocal Linescan" -> [_ _]
      frame #0 {
      }
      frame #1 {
        w1824 = TRUE
        n201 = case shown="True" "Restart DMA? (MCL)" {
          tunnel: [w2068 w2070] -> w1829
          tunnel: [w2067 w2069] -> w1828
          tunnel: w1831 -> [w2068 w2073]
          tunnel: w1830 -> [w2067 w2072]
          frame #0 {
          }
          frame #1 {
            n202 = call "reset FPGA DMA.vi"("error in"=w2072, "FPGA VI Reference In"=w2073) -> ("error out"=w2069:errorcluster, "FPGA VI Reference Out"=w2070:T21)
            n203 = local write "Overflow (data lost)"(FALSE ("Overflow (data lost)")) -> ()
          }
        }
        n204 = case shown="False" w1819 {
          selector: w1819 -> [_ w1835]
          tunnel: w1818 -> [w1834 _]
          tunnel: [w1834 w1835] -> w1817
          frame #0 {
            n205 = property on="2D or 1D Scan" class="Bool (strict)"("Val(Sgnl)"=w1834) -> ()  [unwired: 2 in, 2 out]
            n206 = property on="Confocal Image" class="Bool (strict)"("Value"=FALSE ("Start Confocal Map")) -> ()  [unwired: 2 in, 2 out]
          }
          frame #1 {
          }
        }
        n207 = local write "MCL Scanning"(w1824) -> ()
        n208 = local read "AO1"() -> (w1821:dbl)
        n209 = local read "AO2"() -> (w1820:dbl)
        n210 = case shown="True" "Center Scan" {
          tunnel: w1829 -> [w1842 w1951]
          tunnel: w1828 -> [w1841 w1950]
          tunnel: [w1840 w1949] -> w1826
          tunnel: [w1839 w1948] -> w1825
          tunnel: [w1837 w1935] -> w1823
          tunnel: [w1836 w1934] -> w1822
          tunnel: w1821 -> [w1837 w1940]
          tunnel: w1820 -> [w1836 w1943]
          tunnel: w1817 -> [_ _]
          frame #0 {
            w1838 = TRUE ("AI to FIFO")
            n211 = xnode "Read/Write Control"("FPGA VI Reference In"=w1842, "error in"=w1841, "AI to FIFO"=w1838, "APD to FIFO"=w1838, "Start scan (MCL)"=w1838) -> ("FPGA VI Reference Out"=w1840:T21, "error out"=w1839:errorcluster)
          }
          frame #1 {
            w1947 = TRUE ("AI to FIFO")
            n212 = local read "Scan steps (MCL)"() -> (w1926:u64)
            n213 = local read "Scan lines (y)"() -> (w1922:u64)
            n214 = local read "Fast Scan Dir"() -> (w1933:bool)
            n215 = local read "Actual MCL Inc (V)"() -> (w1923:dbl)
            n216 = Decrement(x=w1922) -> (x-1=w1921:u64)
            n217 = Decrement(x=w1926) -> (x-1=w1925:u64)
            n218 = Multiply(x=w1923, y=w1921) -> (x*y=w1920:dbl)
            n219 = Divide(x=w1920, y=2.0) -> (x/y=w1930:dbl)
            n220 = Multiply(x=w1923, y=w1925) -> (x*y=w1924:dbl)
            n221 = Divide(x=w1924, y=2.0) -> (x/y=w1929:dbl)
            n222 = Select(t=w1929, s=w1933, f=w1930) -> (s? t:f=w1928:dbl)
            n223 = Select(t=w1930, s=w1933, f=w1929) -> (s? t:f=w1932:dbl)
            n224 = Subtract(x=w1940, y=w1932) -> (x-y=w1931:dbl)
            n225 = Subtract(x=w1943, y=w1928) -> (x-y=w1927:dbl)
            n226 = local read "2D or 1D Scan"() -> (w1945:bool)
            n227 = Not(x=w1933) -> (.not. x?=w1939:bool)
            n228 = Not(x=w1945) -> (.not. x?=w1941:bool)
            n229 = And(x=w1933, y=w1941) -> (x .and. y?=w1942:bool)
            n230 = And(x=w1941, y=w1939) -> (x .and. y?=w1944:bool)
            n231 = Select(t=w1943, s=w1944, f=w1927) -> (s? t:f=w1934:dbl)
            n232 = Select(t=w1940, s=w1942, f=w1931) -> (s? t:f=w1935:dbl)
            n233 = call "Volt to I16.vi"("Voltage In"=w1935) -> ("I16 Voltage Out"=w1938:i16)
            n234 = call "Volt to I16.vi"("Voltage In"=w1934) -> ("I16 Voltage Out"=w1937:i16)
            n235 = xnode "Read/Write Control"("FPGA VI Reference In"=w1951, "error in"=w1950, "AI to FIFO"=w1947, "APD to FIFO"=w1947, "Start scan (MCL)"=w1947, "AO1"=w1938, "AO2"=w1937) -> ("FPGA VI Reference Out"=w1949:T21, "error out"=w1948:errorcluster)
          }
        }
        "Initial Y" <- w1823
        "Initial X" <- w1822
        "wait to reset values" <- w1824
      }
    }
    n236 = local read "Trap Pos Elements/DMA read"() -> (w790:u32)
    n237 = local read "Trap AI Elements/DMA read"() -> (w875:u32)
    n238 = local read "APD Elements/DMA read"() -> (w835:u32)
    n239 = xnode "Get APD Data"("FPGA VI Reference In"=w794, "error in"=w793, "Number of Elements"=w835, "Timeout (ms)"=-1) -> ("Data"=w834:u32[], "Elements Remaining"=→"APD FIFO Elements Remaining":u32)  [unwired: 2 out]
    n240 = xnode "Invoke Method"("FPGA VI Reference In"=w794, "error in"=w793, "Number of Elements"=w790, "Timeout (ms)"=-1) -> ("Data"=w753:u16[], "Elements Remaining"=→"Trap Pos FIFO El Remaining":u32)  [unwired: 2 out]
    n241 = xnode "Get Trap Data"("FPGA VI Reference In"=w794, "error in"=w793, "Number of Elements"=w875, "Timeout (ms)"=-1 ("Timeout")) -> ("FPGA VI Reference Out"=w864:T21, "error out"=w863:errorcluster, "Data"=w754:i16[], "Elements Remaining"=w1010:u32)
    "FIFO El. Rem." <- w1010
    n242 = local read "Trap AI FIFO Depth"() -> (w1012:u32)
    n243 = Subtract(x=w1012, y=w875) -> (x-y=w1011:u32)
    n244 = Decimate 1D Array(w753) -> (w750:u16[], w752:u16[], w751:u16[])
    n245 = Divide(x=w1010, y=w1011) -> (x/y=w1009:dbl)
    "Buffer Status" <- w1009
    n246 = To Unsigned Long Integer(number=w750) -> (unsigned 32bit integer=w749:u32[])
    n247 = Join Numbers(hi=w752, lo=w751) -> ((hi.lo)=w748:u32[])
    n248 = Equal?(x=w1009, y=1.0) -> (x = y?=w1007:bool)
    n249 = Join Numbers(hi=w749, lo=w748) -> ((hi.lo)=w742:u64[])
    n250 = call "IR AOM word to freq - vec.vi"("Frequency Word In (double vec)"=w742) -> ("Frequency Out"=w789:dbl[])
    n251 = case "Alert buffer overflow" shown="True" w1007 {
      frame #0 {
      }
      frame #1 {
        n252 = call <vilib>:"Beep.vi"() -> ()  [unwired: 3 in, 9 out]
        "Overflow (data lost)" <- TRUE ("Overflow (data lost)")
      }
    }
    n253 = Decimate 1D Array(w789) -> (w788:dbl[], w787:dbl[])
    n254 = Build Array(w788, w787) -> (w786:dbl[][])
    n255 = local read "Trap Sets"() -> (w874:u32)
    n256 = case "Deinterlace trap data, average down PSD" shown="2" w874 {
      tunnel: w754 -> [w2103 w2168]
      tunnel: [w2100 w2165] -> w867
      tunnel: [w2103 w2167] -> w745
      tunnel: "Detector Type" -> [w2102 w2163]
      tunnel: [w2101 w2166] -> w866
      tunnel: [w2099 w2164] -> w982
      frame #0 {
        n257 = Divide(x=w2103, y=3276.7) -> (x/y=w2104:dbl[])
        n258 = Decimate 1D Array(w2104) -> (w2113:dbl[], w2112:dbl[], w2111:dbl[], w2110:dbl[], w2109:dbl[], w2108:dbl[], w2107:dbl[], w2106:dbl[])
        n259 = case shown="\"IR-QPD + PSD + FB-QPD position\"" w2102 {
          tunnel: w2113 -> [w2137 w2162]
          tunnel: w2112 -> [w2136 w2161]
          tunnel: w2111 -> [w2121 w2139]
          tunnel: w2110 -> [w2122 w2149]
          tunnel: w2109 -> [w2135 w2160]
          tunnel: w2108 -> [w2134 w2159]
          tunnel: w2107 -> [w2118 w2140]
          tunnel: w2106 -> [w2117 w2138]
          tunnel: [w2116 w2146] -> w2101
          tunnel: [w2115 w2145] -> w2100
          tunnel: [w2114 w2144] -> w2099
          frame #0 {
            w2114 = 0  # Channel pattern
            n260 = Divide(x=w2137, y=w2122) -> (x/y=w2124:dbl[])
            n261 = Divide(x=w2136, y=w2122) -> (x/y=w2123:dbl[])
            n262 = Divide(x=w2135, y=w2118) -> (x/y=w2120:dbl[])
            n263 = Divide(x=w2134, y=w2117) -> (x/y=w2119:dbl[])
            n264 = Build Array(w2124, w2123, w2122, w2121, w2120, w2119, w2118, w2117) -> (w2115:dbl[][])
            n265 = Bundle("T1 Y", "T1 X", "T1 Sum", "FB Sum", "PSD Y", "PSD X", "PSD Y Sum", "PSD X Sum") -> (w2133:T35)  [unwired: 1 out]
            n266 = Cluster To Array(cluster=w2133) -> (array=w2116:string[])
          }
          frame #1 {
            w2144 = 3  # Channel pattern
            n267 = Negate(x=w2140) -> (-x=w2141:dbl[])
            n268 = Divide(x=w2162, y=w2149) -> (x/y=w2151:dbl[])
            n269 = Divide(x=w2161, y=w2149) -> (x/y=w2150:dbl[])
            n270 = Divide(x=w2160, y=w2140) -> (x/y=w2148:dbl[])
            n271 = Divide(x=w2159, y=w2141) -> (x/y=w2147:dbl[])
            n272 = Build Array(w2151, w2150, w2149, w2138, w2139, w2148, w2147, w2140) -> (w2145:dbl[][])
            n273 = Bundle("T1 Y", "T1 X", "T1 Sum", "FB X", "FB Sum", "PSD Y", "PSD X", "PSD Y Sum") -> (w2158:T35)  [unwired: 1 out]
            n274 = Cluster To Array(cluster=w2158) -> (array=w2146:string[])
          }
        }
      }
      frame #1 {
        n275 = case shown="\"IR-QPD + PSD + FB-QPD X position\"" w2163 {
          tunnel: w2168 -> [w2230 w2297 w2368]
          tunnel: [w2169 w2288 w2299] -> w2167
          tunnel: [w2196 w2279 w2346] -> w2166
          tunnel: [w2195 w2242 w2313] -> w2165
          tunnel: [w2189 w2277 w2344] -> w2164
          frame #0 {
            w2189 = 1  # Channel pattern
            # "time average x2 the 4th signal and the 4 psd signals (detection laser)"
            # "deinterlace 3 signals from qpd"
            n276 = Decimate 1D Array(w2230) -> (w2229:i16[], w2228:i16[], w2194:i16[], w2227:i16[], w2217:i16[], w2215:i16[], w2214:i16[], w2212:i16[])
            n277 = Decimate 1D Array(w2194) -> (w2193:i16[], w2192:i16[])
            n278 = Decimate 1D Array(w2229) -> (w2226:i16[], w2198:i16[])
            n279 = Decimate 1D Array(w2228) -> (w2225:i16[], w2223:i16[])
            n280 = Decimate 1D Array(w2227) -> (w2224:i16[], w2222:i16[])
            n281 = call "downsample 1D array - double.vi"("Ave N"=2.0, "Array In"=w2217) -> ("Array Out"=w2216:dbl[])  [unwired: 1 out]
            n282 = call "downsample 1D array - double.vi"("Ave N"=2.0, "Array In"=w2215) -> ("Array Out"=w2197:dbl[])  [unwired: 1 out]
            n283 = call "downsample 1D array - double.vi"("Ave N"=2.0, "Array In"=w2214) -> ("Array Out"=w2213:dbl[])  [unwired: 1 out]
            n284 = call "downsample 1D array - double.vi"("Ave N"=2.0, "Array In"=w2212) -> ("Array Out"=w2211:dbl[])  [unwired: 1 out]
            n285 = Interleave 1D Arrays(w2226, w2225, w2224, w2198, w2223, w2222, w2193, w2192, w2216, w2197, w2213, w2211) -> (w2210:dbl[])
            n286 = Divide(x=w2210, y=3276.7) -> (x/y=w2209:dbl[])
            n287 = Decimate 1D Array(w2209) -> (w2208:dbl[], w2207:dbl[], w2206:dbl[], w2205:dbl[], w2204:dbl[], w2203:dbl[], w2191:dbl[], w2190:dbl[], w2202:dbl[], w2201:dbl[], w2200:dbl[], w2199:dbl[])
            n288 = Divide(x=w2208, y=w2206) -> (x/y=w2176:dbl[])
            n289 = Divide(x=w2207, y=w2206) -> (x/y=w2175:dbl[])
            n290 = Divide(x=w2205, y=w2203) -> (x/y=w2174:dbl[])
            n291 = Divide(x=w2204, y=w2203) -> (x/y=w2173:dbl[])
            n292 = Divide(x=w2202, y=w2200) -> (x/y=w2172:dbl[])
            n293 = Divide(x=w2201, y=w2199) -> (x/y=w2171:dbl[])
            n294 = Build Array(w2176, w2175, w2206, w2174, w2173, w2203, w2191, w2190, w2172, w2171, w2200, w2199) -> (w2195:dbl[][])